vi "air mod.vi"() -> ()   [LabVIEW 2018]
panel:
  in  "Tab Control":T1(tab)
  in  "Numeric 3":dbl
  in  "Numeric":dbl
  out "fan":dbl(slide) scale=0.0..10.0
  in  "temp-":bool
  in  "temp+":bool
  out "7 2":bool
  out "6 2":bool
  out "5 2":bool
  out "4 2":bool
  out "1 2":bool
  out "7":bool
  out "6":bool
  out "4":bool
  out "3":bool
  out "1":bool
  in  "TIMER":bool
  in  "Bio sleep":bool
  in  "Auto clean":bool
  in  "Turbo":bool
  in  "Mode":bool
  in  "swing":bool
  in  "on/off":bool
  in  "fan-":bool
  in  "fan+":bool
  in  "Numeric 2":dbl
  # "TEMP"
  # "FAN"
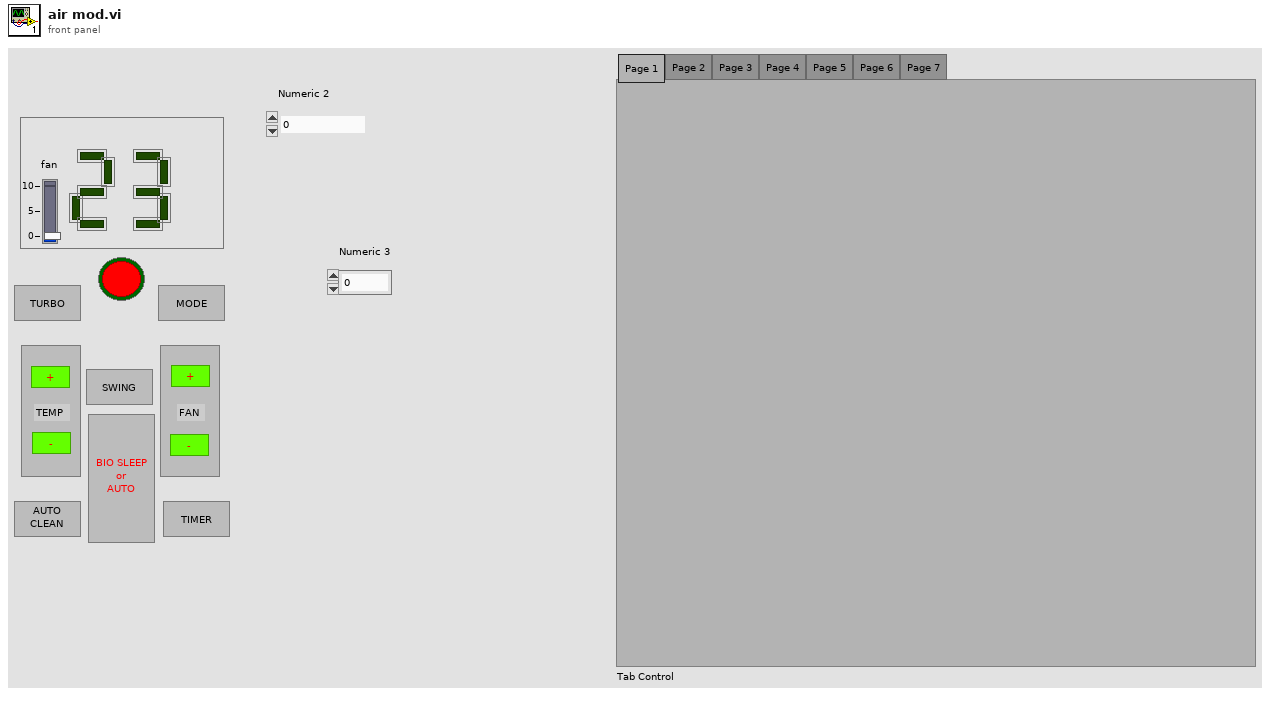
[diagram p1: front panel]
types:
  T1 = enum32{"Page 1", "Page 2", "Page 3", "Page 4", "Page 5", "Page 6", "Page 7"}
  T2 = enum32{"Page 1", "Page 2", "Page 3", "Page 4", "Page 5"}
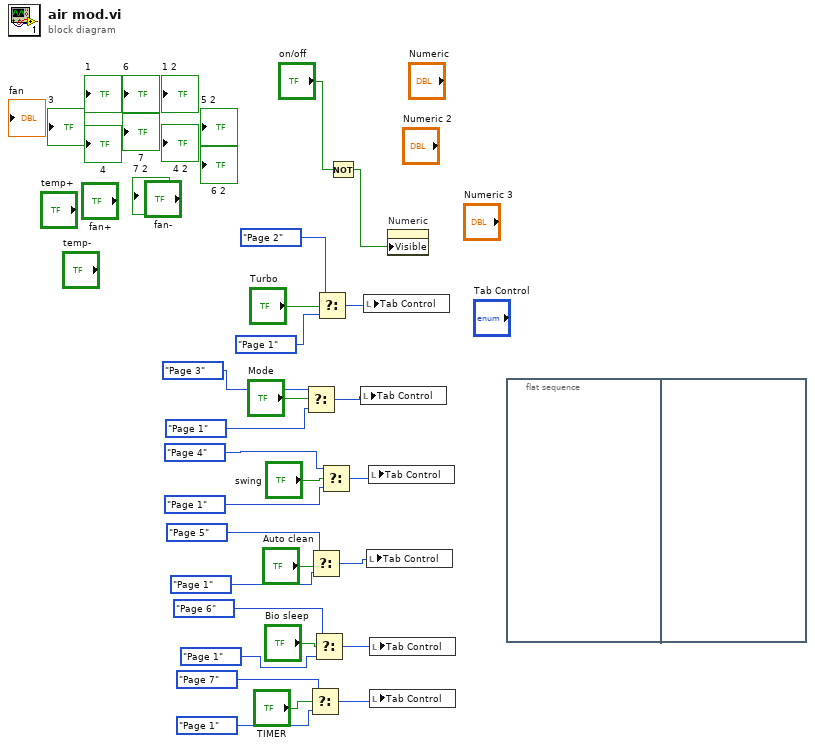
[diagram p0: block diagram]
diagram:
  n1 = Select(t=T2."Page 3" ("Tab Control"), s="Mode", f=enum32{"Page 1", "Page 2"}."Page 1" ("Tab Control")) -> (s? t:f=w10:T2)
  n2 = Select(t=T1."Page 7" ("Tab Control"), s="TIMER", f=enum32{"Page 1", "Page 2"}."Page 1" ("Tab Control")) -> (s? t:f=w6:T1)
  n3 = Select(t=T2."Page 5" ("Tab Control"), s="Auto clean", f=enum32{"Page 1", "Page 2"}."Page 1" ("Tab Control")) -> (s? t:f=w8:T2)
  n4 = Select(t=T1."Page 6" ("Tab Control"), s="Bio sleep", f=enum32{"Page 1", "Page 2"}."Page 1" ("Tab Control")) -> (s? t:f=w7:T1)
  n5 = Select(t=enum32{"Page 1", "Page 2"}."Page 2" ("Tab Control"), s="Turbo", f=enum32{"Page 1", "Page 2"}."Page 1" ("Tab Control")) -> (s? t:f=w22:enum32{"Page 1", "Page 2"})
  n6 = Select(t=T2."Page 4" ("Tab Control"), s="swing", f=enum32{"Page 1", "Page 2"}."Page 1" ("Tab Control")) -> (s? t:f=w9:T2)
  n7 = Not(x="on/off") -> (.not. x?=w25:bool)
  n8 = local write "Tab Control"(w10) -> ()
  n9 = local write "Tab Control"(w22) -> ()
  n10 = local write "Tab Control"(w8) -> ()
  n11 = local write "Tab Control"(w9) -> ()
  n12 = local write "Tab Control"(w7) -> ()
  n13 = local write "Tab Control"(w6) -> ()
  n14 = property on="Numeric" class="DigNum (strict)"("Visible"=w25) -> ()  [unwired: 2 in, 2 out]
  n15 = flat-sequence {
    frame #0 {
    }
    frame #1 {
    }
  }
